vi "UHR-Fleezers Control (host) - 12.7.vi"() -> ()   [LabVIEW 2012] (continued)
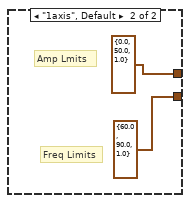
[diagram p2: hidden frame]
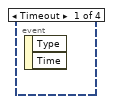
[diagram p3: hidden frame]
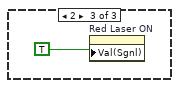
[diagram p6: hidden frame]
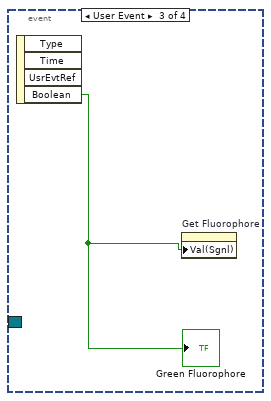
[diagram p7: hidden frame]
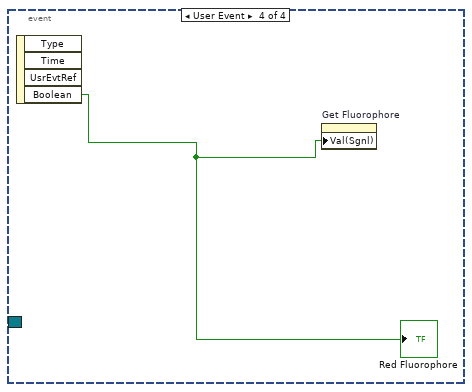
[diagram p8: hidden frame]
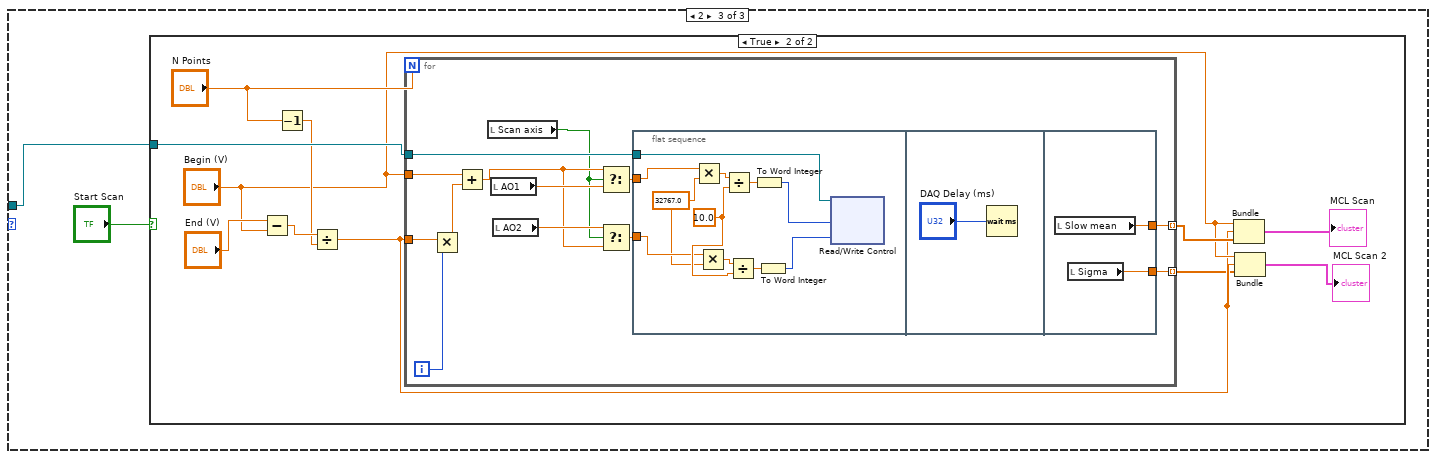
[diagram p10: hidden frame]
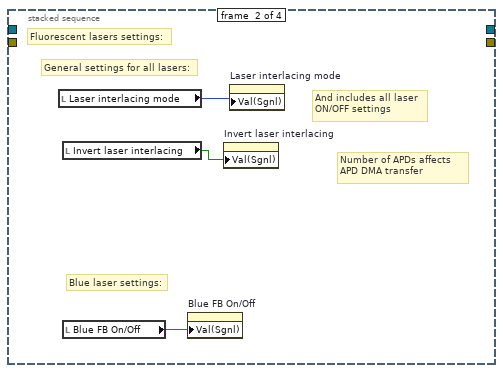
[diagram p12: hidden frame]
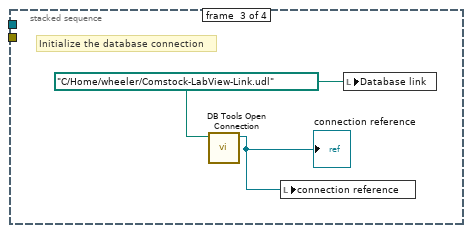
[diagram p13: hidden frame]
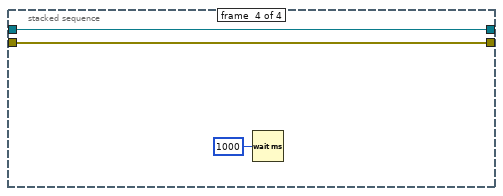
[diagram p14: hidden frame]
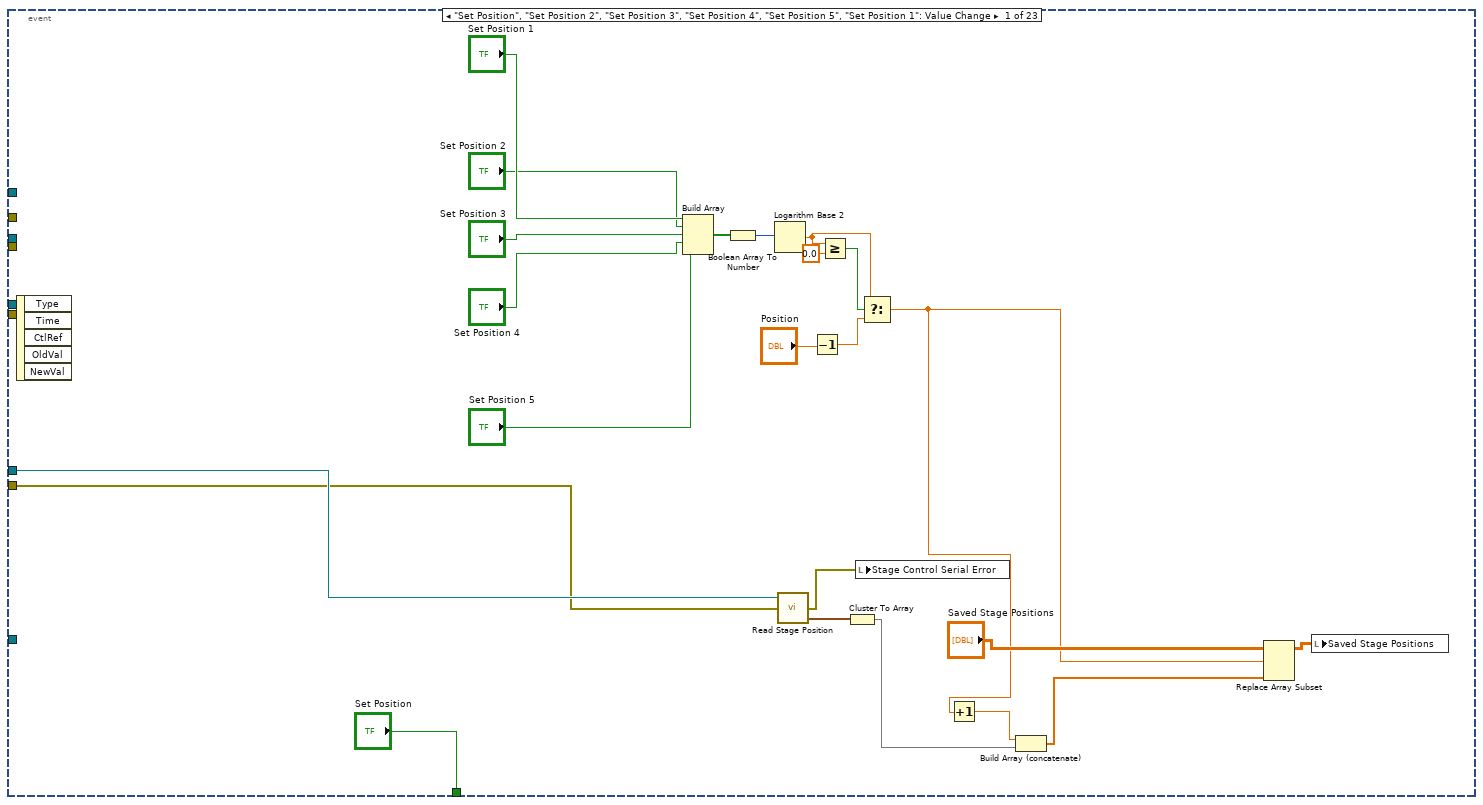
[diagram p16: hidden frame]
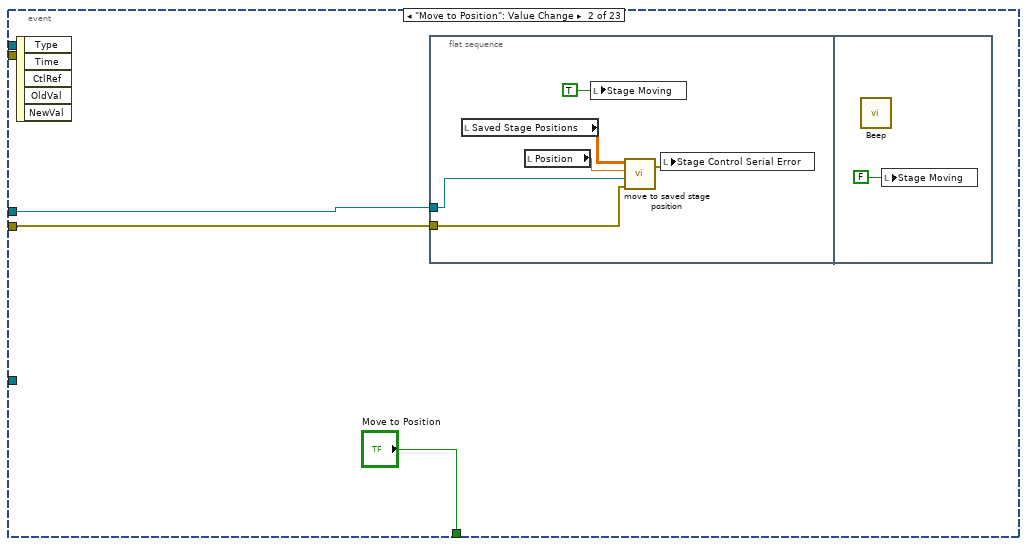
[diagram p17: hidden frame]
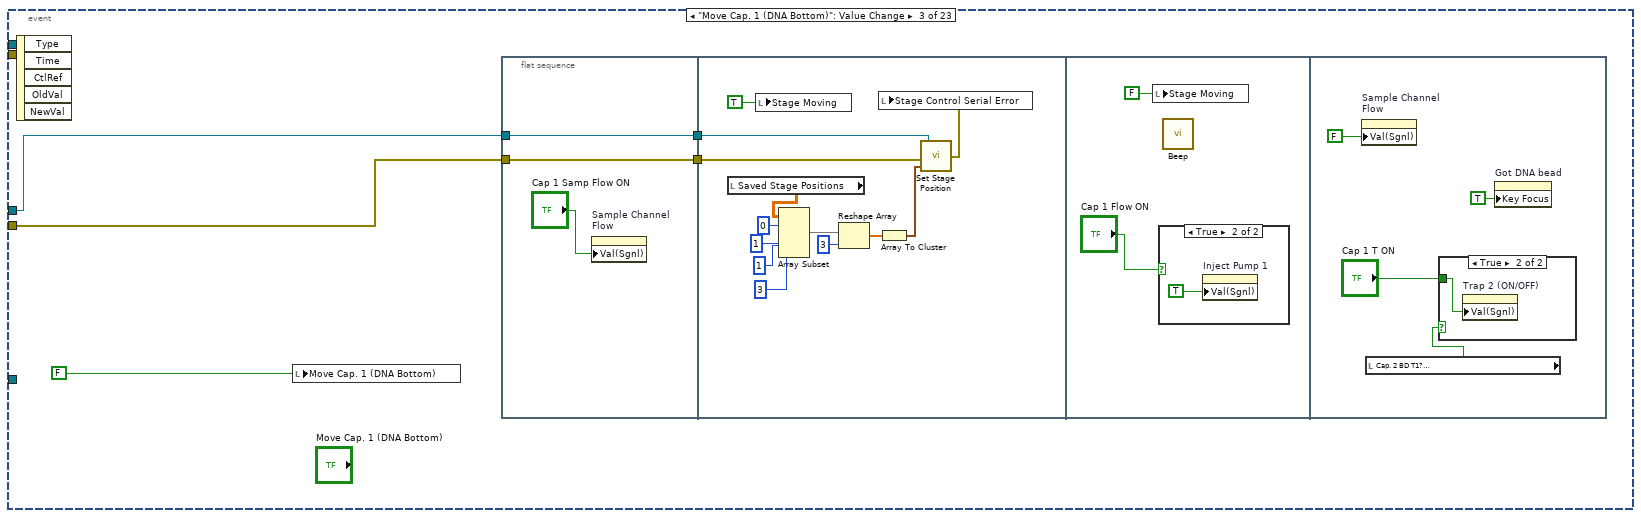
[diagram p18: hidden frame]
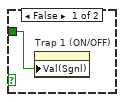
[diagram p20: hidden frame]
              tunnel: [refnum<k0> refnum w4586] -> w4529
              frame False {
              }
              frame True {
                w4585 = 0.0
                n2952 = local read "APD Integration Time (s)"() -> (w4591:dbl)
                n2953 = local read "N APD Samp/step"() -> (w4584:dbl)
                n2954 = local read "Number of APDs"() -> (w4583:u8)
                n2955 = Path To String(path=w4606) -> (string=w4605:string)
                n2956 = String Length(string=w4605) -> (length=w4604:i32)
                n2957 = Subtract(x=w4604, y=4) -> (x-y=w4602:i32)
                n2958 = String Subset(string=w4605, length (rest)=w4602) -> (substring=w4601:string)  [unwired: 1 out]
                n2959 = Build Array(w4591, w4584, w4583, w4585, w4585, w4585, w4585, w4585) -> (w4588:dbl[])
                n2960 = Concatenate Strings(w4601, "_fl.dat" ("string")) -> (w4599:string)
                n2961 = Array Size(array=w4588) -> (size(s)=w4590:i32)
                n2962 = String To Path(string=w4599) -> (path=w4595:path)
                n2963 = Open/Create/Replace File(file path (use dialog)=w4595, operation (0:open)=T29."create", access (0:read/write)=enum16{"read/write", "read-only", "write-only"}."write-only") -> (refnum out=w4596:refnum<file>)  [unwired: 1 in, 4 out]
                n2964 = Deny Access(7:w4596) -> (3:w4592:refnum<file>)  [unwired: 1 in, 2 out]
                n2965 = To Double Precision Float(number=w4590) -> (double precision float=w4589:dbl)
                n2966 = Build Array (concatenate)(w4589, w4588) -> (w4587:dbl[])
                n2967 = Write to Binary File(file (use dialog)=w4592, data=w4587, 5:FALSE ("prepend array or string size? (T)"), 9:T28."big-endian, network order" ("byte order (0:big-endian, network order)")) -> (refnum out=w4586:refnum<file>)  [unwired: 1 in, 3 out]
              }
            }
            n2968 = case shown="True" w4516 {
              tunnel: w4512 -> [_ w4567]
              tunnel: [refnum<k0> refnum w4566] -> w4517
              frame False {
              }
              frame True {
                w4562 = 0.0 ("element")
                n2969 = Path To String(path=w4567) -> (string=w4581:string)
                n2970 = Build Array(w4562, w4562, w4562, w4562, w4562, w4562, w4562, w4562) -> (w4563:dbl[])
                n2971 = String Length(string=w4581) -> (length=w4580:i32)
                n2972 = Subtract(x=w4580, y=4) -> (x-y=w4578:i32)
                n2973 = Array Size(array=w4563) -> (size(s)=w4565:i32)
                n2974 = String Subset(string=w4581, length (rest)=w4578) -> (substring=w4577:string)  [unwired: 1 out]
                n2975 = To Double Precision Float(number=w4565) -> (double precision float=w4564:dbl)
                n2976 = Concatenate Strings(w4577, "_pos.dat" ("string")) -> (w4575:string)
                n2977 = Build Array (concatenate)(w4564, w4563) -> (w4561:dbl[])
                n2978 = String To Path(string=w4575) -> (path=w4571:path)
                n2979 = Open/Create/Replace File(file path (use dialog)=w4571, operation (0:open)=T29."create", access (0:read/write)=enum16{"read/write", "read-only", "write-only"}."write-only") -> (refnum out=w4572:refnum<file>)  [unwired: 1 in, 4 out]
                n2980 = Deny Access(7:w4572) -> (3:w4568:refnum<file>)  [unwired: 1 in, 2 out]
                n2981 = Write to Binary File(file (use dialog)=w4568, data=w4561, 5:FALSE ("prepend array or string size? (T)"), 9:T28."big-endian, network order" ("byte order (0:big-endian, network order)")) -> (refnum out=w4566:refnum<file>)  [unwired: 1 in, 3 out]
              }
            }
            n2982 = Write to Binary File(file (use dialog)=w4552, data=w4511, 5:w4534, 9:w4533) -> (refnum out=w4535:refnum<file>)  [unwired: 1 in, 3 out]
            n2983 = Write to Binary File(file (use dialog)=w4535, data="Comment (data description)", 5:w4534, 9:w4533) -> (refnum out=w4532:refnum<file>)  [unwired: 1 in, 3 out]
            n2984 = local read "connection reference"() -> (w4514:T17)
            n2985 = Bundle("Comment (data description)"="Comment (data description)", "Channel 1 Buffer"="Channel 1 Buffer", "Channel 2 Buffer"="Channel 2 Buffer", "Channel 3 Buffer"="Channel 3 Buffer", "Title"="Title", "DNA Construct"="DNA Construct", "Bead diameter"="Bead diameter", "Name"="Name") -> (w4502:T47)  [unwired: 1 in]
            n2986 = call "MattFileCreator-v9.vi"("Comments"=w4502, "Input Array"=w4511, "File path"=w4512, "table"="labview", "connection reference"=w4514) -> ("connection reference out"=w4513:T17)  [unwired: 5 in, 1 out]
            n2987 = local write "connection reference"(w4513) -> ()
          }
        }
        n2988 = feedback-in #27(w4462) -> ()
        n2989 = feedback-in #28(w4489) -> ()
        n2990 = feedback-in #29(w4461) -> ()
        n2991 = feedback-in #30(w4472) -> ()
        n2992 = feedback-in #31(w4475) -> ()
        n2993 = feedback-in #32(w4488) -> ()
        n2994 = feedback-in #33(w4478) -> ()
      }
      frame #1 {
        n2995 = local read "Saving..."() -> (w4732:bool)
        n2996 = case shown="True" w4732 {
          tunnel: w4736 -> [_ w4747]
          tunnel: w4735 -> [_ w4761]
          tunnel: w4734 -> [_ w4757]
          tunnel: w4733 -> [_ w4756]
          tunnel: w4731 -> [_ w4755]
          tunnel: w4730 -> [_ w4750]
          tunnel: w4729 -> [_ w4749]
          tunnel: w4728 -> [_ w4748]
          tunnel: w4727 -> [_ w4746]
          tunnel: w4726 -> [_ w4744]
          tunnel: w4725 -> [_ w4743]
          tunnel: w4724 -> [_ w4742]
          tunnel: w4723 -> [_ w4741]
          tunnel: w4722 -> [_ w4740]
          tunnel: w4721 -> [_ w4739]
          tunnel: w4720 -> [_ w4738]
          tunnel: w4719 -> [_ w4737]
          frame False {
          }
          frame True {
            n2997 = Multiply(x=w4747, y=w4746) -> (x*y=→"Time (s)":dbl)
            n2998 = Less Or Equal?(x=w4747, y=w4755) -> (x <= y?=w4759:bool)
            n2999 = Or(x="Stop Saving", y="Abort save 2") -> (x .or. y?=w4751:bool)
            n3000 = Not(x=w4751) -> (.not. x?=w4760:bool)
            n3001 = And(x=w4759, y=w4760) -> (x .and. y?=w4758:bool)
            n3002 = case shown="True" w4758 {
              tunnel: w4761 -> [w4768 w4859]
              tunnel: [0.0 w4862] -> w4754
              tunnel: w4747 -> [_ w4860]
              tunnel: w4755 -> [_ w4861]
              tunnel: w4757 -> [_ w4856]
              tunnel: w4756 -> [_ _]
              tunnel: w4750 -> [w4766 w4849]
              tunnel: w4749 -> [w4765 w4850]
              tunnel: w4748 -> [_ w4848]
              tunnel: w4744 -> [_ w4847]
              tunnel: w4743 -> [_ w4771]
              tunnel: w4742 -> [_ w4840]
              tunnel: w4741 -> [_ w4787]
              tunnel: w4740 -> [w4762 w4804]
              tunnel: w4739 -> [w4763 w4803]
              tunnel: w4738 -> [_ w4800]
              tunnel: w4737 -> [_ w4798]
              frame False {
                w4764 = FALSE
                n3003 = Close File(refnum=w4768) -> ()  [unwired: 1 in, 2 out]
                n3004 = case shown="True" w4765 {
                  tunnel: w4766 -> [_ w4770]
                  frame False {
                  }
                  frame True {
                    n3005 = Close File(refnum=w4770) -> ()  [unwired: 1 in, 2 out]
                  }
                }
                n3006 = case shown="True" w4762 {
                  tunnel: w4763 -> [_ w4769]
                  frame False {
                  }
                  frame True {
                    n3007 = Close File(refnum=w4769) -> ()  [unwired: 1 in, 2 out]
                  }
                }
                n3008 = local write "Raster Scanning..."(w4764) -> ()
                n3009 = local write "Calibrating Trap..."(w4764) -> ()
                n3010 = call <vilib>:"Beep.vi"() -> ()  [unwired: 3 in, 9 out]
                n3011 = local write "Stop Saving"(w4764) -> ()
                "Saving..." <- w4764
              }
              frame True {
                n3012 = local read "Calibrating Trap..."() -> (w4851:bool)
                n3013 = case "Write fl. data" shown="True" w4850 {
                  tunnel: w4849 -> [_ w4885]
                  tunnel: w4848 -> [_ w4884]
                  frame False {
                  }
                  frame True {
                    n3014 = Write to Binary File(file (use dialog)=w4885, data=w4884, 5:FALSE ("prepend array or string size? (T)"), 9:T28."big-endian, network order" ("byte order (0:big-endian, network order)")) -> ()  [unwired: 1 in, 4 out]
                  }
                }
                n3015 = Greater?(x="Save ave N", y=1.0) -> (0:w4854:bool)
                n3016 = Not(x=w4851) -> (.not. x?=w4853:bool)
                n3017 = And(x=w4853, y=w4854) -> (x .and. y?=w4801:bool)
                n3018 = case shown="True" w4801 {
                  tunnel: w4800 -> [w4865 w4876]
                  tunnel: [w4865 w4868] -> w4799
                  tunnel: "Save ave N" -> [_ w4869]
                  frame False {
                  }
                  frame True {
                    w4866 = 2 ("dimension size")
                    n3019 = Array Size(array=w4876) -> (size(s)=w4870:i32)
                    n3020 = Divide(x=w4870, y=w4866) -> (x/y=w4874:dbl)
                    n3021 = Reshape Array(w4876, w4874, w4866) -> (w4875:u64[][])
                    n3022 = Transpose 2D Array(2D array=w4875) -> (transposed array=w4873:u64[][])
                    n3023 = for {
                      tunnel: w4873 -> [w4878] mode=indexing
                      tunnel: [w4877] -> w4867 mode=indexing
                      tunnel: w4869 -> [w4879]
                      workers-P: _ -> [_]
                      n3024 = call "downsample 1D array - U64.vi"("Ave N"=w4879, "Array In"=w4878) -> ("Array Out"=w4877:u64[])  [unwired: 1 in]
                    }
                    n3025 = Transpose 2D Array(2D array=w4867) -> (transposed array=w4872:u64[][])
                    n3026 = Divide(x=w4870, y=w4869) -> (x/y=w4871:dbl)
                    n3027 = Reshape Array(w4872, w4871) -> (w4868:u64[])
                  }
                }
                n3028 = case shown="True" w4801 {
                  tunnel: w4856 -> [w4888 w4900]
                  tunnel: [w4888 w4892] -> w4852
                  tunnel: "Save ave N" -> [_ w4893]
                  tunnel: w4847 -> [_ w4891]
                  frame False {
                  }
                  frame True {
                    n3029 = Array Size(array=w4900) -> (size(s)=w4894:i32)
                    n3030 = Array Size(array=w4891) -> (size(s)=w4890:i32)
                    n3031 = Divide(x=w4894, y=w4890) -> (x/y=w4898:dbl)
                    n3032 = Reshape Array(w4900, w4898, w4890) -> (w4899:i16[][])
                    n3033 = Transpose 2D Array(2D array=w4899) -> (transposed array=w4897:i16[][])
                    n3034 = for {
                      tunnel: w4897 -> [w4903] mode=indexing
                      tunnel: [w4902] -> w4889 mode=indexing
                      tunnel: w4893 -> [w4901]
                      workers-P: _ -> [_]
                      n3035 = call "downsample 1D array - I16.vi"("Ave N"=w4901, "Array In"=w4903) -> ("Array Out"=w4902:i16[])  [unwired: 1 out]
                    }
                    n3036 = Transpose 2D Array(2D array=w4889) -> (transposed array=w4896:i16[][])
                    n3037 = Divide(x=w4894, y=w4893) -> (x/y=w4895:dbl)
                    n3038 = Reshape Array(w4896, w4895) -> (w4892:i16[])
                  }
                }
                n3039 = Index Array(array=w4787, index=2) -> (element=w4788:waveform(dbl))
                n3040 = Index Array(array=w4787, index=1) -> (element=w4821:waveform(dbl))
                n3041 = Index Array(array=w4787, index=0) -> (element=w4823:waveform(dbl))
                n3042 = Unbundle By Name(w4788) -> ("Y"=w4790:dbl[])
                n3043 = Unbundle By Name(w4821) -> ("Y"=w4825:dbl[])
                n3044 = Unbundle By Name(w4823) -> ("Y"=w4833:dbl[])
                n3045 = case "Write trap pos. data" shown="True" w4804 {
                  tunnel: w4803 -> [_ w4881]
                  tunnel: w4799 -> [_ w4880]
                  frame False {
                  }
                  frame True {
                    n3046 = Write to Binary File(file (use dialog)=w4881, data=w4880, 5:FALSE ("prepend array or string size? (T)"), 9:T28."big-endian, network order" ("byte order (0:big-endian, network order)")) -> ()  [unwired: 1 in, 4 out]
                  }
                }
                n3047 = Write to Binary File(file (use dialog)=w4859, data=w4852, 5:FALSE ("prepend array or string size? (T)"), 9:T28."big-endian, network order" ("byte order (0:big-endian, network order)")) -> ()  [unwired: 1 in, 4 out]
                n3048 = feedback #34(w4790) -> (w4791:dbl[])
                n3049 = Build Array (concatenate)(w4791, w4790) -> (w4786:dbl[])
                n3050 = Select(t=w4790, s=w4771, f=w4786) -> (s? t:f=w4776:dbl[])
                n3051 = feedback-in #34(w4776) -> ()
                n3052 = feedback #35(w4825) -> (w4827:dbl[])
                n3053 = Build Array (concatenate)(w4827, w4825) -> (w4826:dbl[])
                n3054 = Select(t=w4825, s=w4771, f=w4826) -> (s? t:f=w4815:dbl[])
                n3055 = feedback-in #35(w4815) -> ()
                n3056 = feedback #36(w4833) -> (w4846:dbl[])
                n3057 = Build Array (concatenate)(w4846, w4833) -> (w4845:dbl[])
                n3058 = Select(t=w4833, s=w4771, f=w4845) -> (s? t:f=w4820:dbl[])
                n3059 = feedback-in #36(w4820) -> ()
                n3060 = Divide(x=w4860, y=w4861) -> (x/y=w4863:dbl)
                n3061 = Multiply(x=w4863, y=100.0) -> (x*y=w4862:dbl)
                n3062 = Build Array(w4820, w4815, w4776) -> (→"Saved APD":dbl[][])
                n3063 = Array Size(array=w4820) -> (size(s)=w4838:i32)
                n3064 = Unbundle By Name(w4840) -> ("Y"=w4844:dbl[])
                n3065 = Subtract(x=w4838, y="N pts to average") -> (x-y=w4773:i32)
                n3066 = Multiply(x="N pts to average", y=u16 2) -> (x*y=w4816:u16)
                n3067 = Subtract(x=w4838, y=w4816) -> (x-y=w4774:i32)
                n3068 = feedback #37(w4844) -> (w4843:dbl[])
                n3069 = Build Array (concatenate)(w4843, w4844) -> (w4842:dbl[])
                n3070 = Select(t=w4844, s=w4771, f=w4842) -> (s? t:f=w4841:dbl[])
                "Trap Delta Graph" <- w4841
                n3071 = feedback-in #37(w4841) -> ()
                n3072 = Array Subset(array=w4820, index=w4773, length="N pts to average") -> (w4837:dbl[])
                n3073 = Array Subset(array=w4820, index=w4774, length="N pts to average") -> (w4836:dbl[])
                n3074 = Array Subset(array=w4815, index=w4773, length="N pts to average") -> (w4818:dbl[])
                n3075 = Array Subset(array=w4815, index=w4774, length="N pts to average") -> (w4817:dbl[])
                n3076 = Array Subset(array=w4776, index=w4773, length="N pts to average") -> (w4785:dbl[])
                n3077 = Array Subset(array=w4776, index=w4774, length="N pts to average") -> (w4784:dbl[])
                n3078 = Index Array(array=w4798, index=0) -> (element=w4796:waveform(dbl))
                n3079 = call-poly <vilib>:"Mean.vi"("X"=w4837) -> ("mean"=w4835:dbl)  [unwired: 1 out]
                n3080 = call-poly <vilib>:"Mean.vi"("X"=w4818) -> ("mean"=w4814:dbl)  [unwired: 1 out]
                n3081 = call-poly <vilib>:"Mean.vi"("X"=w4836) -> ("mean"=w4834:dbl)  [unwired: 1 out]
                n3082 = call-poly <vilib>:"Mean.vi"("X"=w4817) -> ("mean"=w4813:dbl)  [unwired: 1 out]
                n3083 = call-poly <vilib>:"Mean.vi"("X"=w4785) -> ("mean"=w4783:dbl)  [unwired: 1 out]
                n3084 = call-poly <vilib>:"Mean.vi"("X"=w4784) -> ("mean"=w4782:dbl)  [unwired: 1 out]
                n3085 = Unbundle By Name(w4796) -> ("Y"=w4794:dbl[])
                n3086 = Subtract(x=w4814, y=w4813) -> (x-y=w4805:dbl)
                "Delta Fl. 2" <- w4805
                n3087 = Subtract(x=w4783, y=w4782) -> (x-y=w4777:dbl)
                "Delta Fl. 3" <- w4777
                n3088 = Subtract(x=w4835, y=w4834) -> (x-y=w4832:dbl)
                "Delta Fl. 1" <- w4832
                n3089 = feedback #38(w4794) -> (w4793:dbl[])
                n3090 = Build Array (concatenate)(w4793, w4794) -> (w4795:dbl[])
                n3091 = Initialize Array(w4832, 1 ("dimension size")) -> (w4829:dbl[])
                n3092 = Initialize Array(w4805, 1 ("dimension size")) -> (w4810:dbl[])
                n3093 = Initialize Array(w4777, 1 ("dimension size")) -> (w4779:dbl[])
                n3094 = Select(t=w4794, s=w4771, f=w4795) -> (s? t:f=w4792:dbl[])
                "Saved trap pos" <- w4792
                n3095 = feedback-in #38(w4792) -> ()
                n3096 = feedback #39(w4829) -> (w4830:dbl[])
                n3097 = Build Array (concatenate)(w4830, w4829) -> (w4828:dbl[])
                n3098 = feedback #40(w4810) -> (w4811:dbl[])
                n3099 = feedback #41(w4779) -> (w4780:dbl[])
                n3100 = Build Array (concatenate)(w4811, w4810) -> (w4809:dbl[])
                n3101 = Build Array (concatenate)(w4780, w4779) -> (w4778:dbl[])
                n3102 = Select(t=w4829, s=w4771, f=w4828) -> (s? t:f=w4808:dbl[])
                n3103 = feedback-in #39(w4808) -> ()
                n3104 = Select(t=w4810, s=w4771, f=w4809) -> (s? t:f=w4807:dbl[])
                n3105 = feedback-in #40(w4807) -> ()
                n3106 = Select(t=w4779, s=w4771, f=w4778) -> (s? t:f=w4772:dbl[])
                n3107 = feedback-in #41(w4772) -> ()
                n3108 = Build Array(w4808, w4807, w4772) -> (→"Save APD Deriv":dbl[][])
              }
            }
            "Progress" <- w4754
            "Progress 2" <- w4754
          }
        }
      }
    }
    n3109 = local read "wait to reset values"() -> (w3406:bool)
    n3110 = Not(x=w3404) -> (.not. x?=w3407:bool)
    n3111 = And(x=w3407, y=w3406) -> (x .and. y?=w3408:bool)
    n3112 = case "Part of MCL raster scanning: returns to initial positions after scan done" shown="True" w3408 {
      tunnel: w3139 -> [w4282 w4289]
      tunnel: [w4282 w4288] -> w3410
      tunnel: w3138 -> [w4281 w4287]
      tunnel: [w4281 w4286] -> w3405
      frame False {
      }
      frame True {
        w4297 = 10.0 ("y")
        w4296 = 32767.0 ("y")
        # "to return scan values\nafter a synchronous \nAOM scan"
        n3113 = local read "AO2"() -> (w4290:dbl)
        n3114 = local read "AO1"() -> (w4291:dbl)
        n3115 = local write "wait to reset values"(FALSE ("wait to reset values")) -> ()
        n3116 = Multiply(x=w4291, y=w4296) -> (x*y=w4293:dbl)
        n3117 = Multiply(x=w4290, y=w4296) -> (x*y=w4295:dbl)
        n3118 = Divide(x=w4293, y=w4297) -> (x/y=w4292:dbl)
        n3119 = Divide(x=w4295, y=w4297) -> (x/y=w4294:dbl)
        n3120 = To Word Integer(number=w4292) -> (16bit integer=w4298:i16)
        n3121 = To Word Integer(number=w4294) -> (16bit integer=w4299:i16)
        n3122 = local read "Total Counts (ticks)"() -> (w4283:u16)
        n3123 = xnode "Read/Write Control"("FPGA VI Reference In"=w4289, "error in"=w4287, "AO1"=w4298, "AO2"=w4299, "MCL count"=w4283) -> ("FPGA VI Reference Out"=w4288:T20, "error out"=w4286:errorcluster)
        n3124 = local read "Scan Range (V)\n(of steps)"() -> (w4284:dbl)
        n3125 = property on="Scan Range (V)\n(of steps)" class="DigNum (strict)"("Val(Sgnl)"=w4284) -> ()  [unwired: 2 in, 2 out]
      }
    }
    n3126 = node-c288() -> ()  [unwired: 2 out]
  }
  n3127 = flat-sequence "Video" {
    tunnel: [w4913] -> w116
    tunnel: w116 -> [w4953]
    frame #0 {
      n3128 = while {
        stop <- w4905 continue-if-true
        n3129 = call "Close Video Capture.vi"() -> ("error code OUT"=w4907:i32)
        n3130 = Equal?(x=w4907, y=0) -> (x = y?=w4905:bool)
      }
      n3131 = local write "Stop All"(FALSE ("Stop All")) -> ()
    }
    frame #1 {
      n3132 = call "DMR_Init.vi"() -> ()  [unwired: 3 out]
    }
    frame #2 {
      w4908 = "DE245428202"  # MSU fleezers card #
      (unwired) "DE019116701"  # Illinois fleezers card #
      # "Setting the destination format to Mono8 makes sure that the image can be displayed in the intensity plot."
      n3133 = call "DMR_GetDevice.vi"("search string IN"=w4908) -> ("device handle OUT"=w4931:i32)  [unwired: 4 in, 2 out]
      n3134 = call "DMR_OpenDevice.vi"("device handle IN"=w4931) -> ("driver handle OUT"=w4914:i32)  [unwired: 4 out]
      n3135 = call "DMR_FindList.vi"("flags IN"=u32 0 ("flags"), "list name IN"="" ("String"), "list type IN"=T48."camera descriptions", "driver handle IN"=w4914) -> ("list handle OUT"=w4917:i32)  [unwired: 2 out]
      n3136 = call "DMR_FindList.vi"("flags IN"=u32 0 ("flags"), "list name IN"="Base", "list type IN"=T48."setting", "driver handle IN"=w4914) -> ("list handle OUT"=w4915:i32)  [unwired: 2 out]
      n3137 = call "OBJ_GetHandle.vi"("object name IN"="VideoStandard", "list handle IN"=w4917) -> ("object handle OUT"=w4911:i32)  [unwired: 3 out]
      n3138 = call "OBJ_GetHandle.vi"("object name IN"="PixelFormat", "list handle IN"=w4915) -> ("object handle OUT"=w4925:i32)  [unwired: 3 out]
      n3139 = call "OBJ_SetS.vi"("value index IN"=0, "value IN"="NTSC M", "object handle IN"=w4911) -> ()  [unwired: 2 out]
      n3140 = call "OBJ_SetS.vi"("value index IN"=0, "value IN"="Mono8" ("value"), "object handle IN"=w4925) -> ()  [unwired: 2 out]
      n3141 = call "OBJ_GetHandle.vi"("object name IN"="VideoChannel", "list handle IN"=w4915) -> ("object handle OUT"=w4921:i32)  [unwired: 3 out]
      n3142 = while {
        tunnel: [w4935] -> w4913
        tunnel: w4914 -> [w4932]
        stop <- w4933 continue-if-true
        n3143 = call "DMR_ImageRequestSingle.vi"("request control IN"=0, "driver handle IN"=w4932) -> ("error code OUT"=w4934:i32, "driver handle OUT"=w4935:i32)  [unwired: 2 out]
        n3144 = Equal To 0?(x=w4934) -> (x = 0?=w4933:bool)
      }
      n3145 = call "OBJ_SetI.vi"("value index IN"=0, "value IN"=3 ("Video channel"), "object handle IN"=w4921) -> ()  [unwired: 2 out]
    }
    frame #3 {
      w4941 = T18 0 items=["Grayscale (U8)", "Grayscale (I16)", "Grayscale (SGL)", "Complex (CSG)", "RGB (U32)", "HSL (U32)", "RGB (U64)"] ("Image Type")
      w4949 = T18 0 items=["Grayscale (U8)", "Grayscale (I16)", "Grayscale (SGL)", "Complex (CSG)", "RGB (U32)", "HSL (U32)", "RGB (U64)"] ("Image Type")
      n3146 = for "Create Greyscale map" {
        N: 256 -> [_]
        tunnel: [w4955] -> w4938 mode=indexing
        workers-P: _ -> [_]
        i -> [w4958]
        n3147 = To Unsigned Byte Integer(number=w4958) -> (unsigned 8bit integer=w4954:u8)
        n3148 = Join Numbers(hi=w4954, lo=w4954) -> ((hi.lo)=w4957:u16)
        n3149 = Join Numbers(hi=w4954, lo=w4954) -> ((hi.lo)=w4956:u16)
        n3150 = Join Numbers(hi=w4957, lo=w4956) -> ((hi.lo)=w4955:u32)
      }
      n3151 = call "IMAQ Create"("Image Name"="Scaled video", "Image Type"=w4941) -> ("New Image"=w4940:T2)  [unwired: 2 in, 2 out]
      n3152 = call "IMAQ Create"("Image Name"="Main video", "Image Type"=w4949) -> ("New Image"=w4950:T2)  [unwired: 2 in, 2 out]
      n3153 = node-c288(0 ("Processor")) -> (w4948:T23)  [unwired: 3 out]
      n3154 = Initialize Array(u32 0 ("Window Number (0...15)"), 480 ("dimension size"), 640 ("dimension size")) -> (w4943:u32[][])
      n3155 = timed-loop {
        tunnel: w4953 -> [w4975]
        tunnel: [w4974] -> w4952
        tunnel: w4950 -> [w4973]
        timing: w4948 -> [_]
        timing-out: [_] -> w4947
        tunnel: w4943 -> [w4962]
        tunnel: w4940 -> [w4960]
        tunnel: w4938 -> [w4959]
        stop <- w4961 stop-if-true
        # "This block performs the \nactual image capture."
        n3156 = node-c288() -> ()  [unwired: 2 out]
        n3157 = local read "Stop All"() -> (w4961:bool)
        n3158 = Reciprocal(x="Video Capture Rate (Hz)") -> (1/x=w4965:dbl)
        n3159 = Multiply(x=w4965, y=1000.0) -> (x*y=w4963:dbl)
        n3160 = call "DMR_ImageRequestWaitFor.vi"("queue number IN"=0, "timeout(ms) IN"=500, "driver handle IN"=w4975) -> ("error code OUT"=w4979:i32, "request number OUT"=w4976:i32, "driver handle OUT"=w4977:i32)
        n3161 = feedback #42(T49 refnum ("Avi Refnum")) -> (w4967:T49)
        n3162 = case shown="True" "New Video File" {
          tunnel: [T49 refnum ("Avi Refnum") w4996] -> w4969
          tunnel: [FALSE TRUE] -> w4970
          tunnel: w4967 -> [_ w4992]
          frame False {
          }
          frame True {
            n3163 = call "Create new save file.vi"("Ext"=".avi" ("string"), "Index In"="Video Index") -> ("Path Out"=w4988:path, "Index Out"=w4989:dbl)  [unwired: 1 in]
            "Path Out" <- w4988
            n3164 = Not Equal?(x=w4992, y=T49 refnum ("Avi Refnum")) -> (x != y?=w4993:bool)
            n3165 = Increment(x=w4989) -> (x+1=w4998:dbl)
            n3166 = case shown="True" w4993 {
              tunnel: w4992 -> [_ w4999]
              frame False {
              }
              frame True {
                n3167 = call "IMAQ AVI Close"("Avi Refnum"=w4999) -> ()  [unwired: 1 in, 10 out]
              }
            }
            n3168 = local write "Video Index"(w4998) -> ()
            n3169 = call "IMAQ AVI Create"("Frames Per Second"=u32 30, "AVI Path"=w4988) -> ("Avi Refnum"=w4996:T49)  [unwired: 5 in, 4 out]
          }
        }
        n3170 = Equal To 0?(x=w4979) -> (x = 0?=w4978:bool)
        n3171 = Select(t=w4969, s=w4970, f=w4967) -> (s? t:f=w4968:T49)
        n3172 = feedback-in #42(w4968) -> ()
        n3173 = case shown="True" w4978 {
          tunnel: w4977 -> [w5000 w5034]
          tunnel: w4976 -> [_ w5033]
          tunnel: [w5000 w5030] -> w4974
          tunnel: w4973 -> [_ w5015]
          tunnel: w4962 -> [_ w5019]
          tunnel: w4968 -> [_ w5017]
          tunnel: w4960 -> [_ w5012]
          tunnel: w4959 -> [_ w5011]
          frame False {
          }
          frame True {
            w5024 = u32 0 ("X-offset IN")
            n3174 = call "DMR_GetImageRequestBufferData.vi"("driver handle IN"=w5034, "request number IN"=w5033) -> ("width OUT"=w5023:i32, "height OUT"=w5022:i32, "driver handle OUT"=w5029:i32, "request number OUT"=w5028:i32, "bytes per pixel OUT"=w5025:i32)  [unwired: 13 out]
            n3175 = call "DMR_GetImageRequestBufferImageData.vi"("driver handle IN"=w5029, "request number IN"=w5028, "bytes per pixel IN"=w5025, "X-offset IN"=w5024, "Y-offset IN"=w5024, "height IN"=w5022, "width IN"=w5023) -> ("driver handle OUT"=w5027:u32, "request number OUT"=w5026:u32, "image OUT"=w5004:u32[][])  [unwired: 10 out]
            n3176 = Transpose 2D Array(2D array=w5004) -> (transposed array=w5010:u32[][])
            n3177 = Select(t=w5010, s="Flip Y (or X)", f=w5004) -> (s? t:f=w5009:u32[][])
            n3178 = call "DMR_ImageRequestUnlock.vi"("request number IN"=w5026, "driver handle IN"=w5027) -> ("driver handle OUT"=w5032:i32)  [unwired: 1 in, 2 out]
            n3179 = for {
              tunnel: w5009 -> [w5069] mode=indexing
              tunnel: [w5068] -> w5007 mode=indexing
              n3180 = Reverse 1D Array(array=w5069) -> (reversed array=w5068:u32[])
            }
            n3181 = call "DMR_ImageRequestSingle.vi"("request control IN"=0, "driver handle IN"=w5032) -> ("driver handle OUT"=w5030:i32)  [unwired: 3 out]
            n3182 = Transpose 2D Array(2D array=w5007) -> (transposed array=w5008:u32[][])
            n3183 = Select(t=w5008, s="Flip Y (or X)", f=w5007) -> (s? t:f=w5005:u32[][])
            n3184 = Select(t=w5005, s="Flip Image", f=w5004) -> (s? t:f=w5002:u32[][])
            n3185 = case shown="True" "Averaging" {
              tunnel: w5002 -> [w5072 w5077]
              tunnel: [w5072 w5076] -> w5016
              tunnel: w5019 -> [_ w5074]
              frame False {
              }
              frame True {
                (unwired) 1
                w5082 = 1
                n3186 = feedback #43(w5074) -> (w5073:u32[][])
                n3187 = Add(x=w5077, y=w5073) -> (x+y=w5078:u32[][])
                n3188 = Select(t=w5074, s="Reset Averaging", f=w5078) -> (s? t:f=w5080:u32[][])
                n3189 = feedback-in #43(w5080) -> ()
                n3190 = feedback #44(w5082) -> (w5075:i32)
                n3191 = Divide(x=w5078, y=w5075) -> (x/y=w5079:dbl[][])
                n3192 = Increment(x=w5075) -> (x+1=w5083:i32)
                n3193 = To Unsigned Long Integer(number=w5079) -> (unsigned 32bit integer=w5076:u32[][])
                n3194 = Select(t=w5082, s="Reset Averaging", f=w5083) -> (s? t:f=w5081:i32)
                n3195 = feedback-in #44(w5081) -> ()
              }
            }
            n3196 = case shown="True" "Zoom video window" {
              tunnel: w5016 -> [_ w5048]
              tunnel: w5012 -> [_ w5047]
              frame False {
              }
              frame True {
                n3197 = To Double Precision Float(number=w5048) -> (double precision float=w5045:dbl[][])
                n3198 = In Range and Coerce(upper limit="Intensity Upper", x=w5045, lower limit="Intensity Lower") -> (coerced(x)=w5044:dbl[][])  [unwired: 1 out]
                n3199 = Subtract(x="Intensity Upper", y="Intensity Lower") -> (x-y=w5041:dbl)
                n3200 = Subtract(x=w5044, y="Intensity Lower") -> (x-y=w5042:dbl[][])
                n3201 = Divide(x=w5042, y=w5041) -> (x/y=w5043:dbl[][])
                n3202 = Multiply(x=255.0, y=w5043) -> (x*y=w5039:dbl[][])
                n3203 = To Unsigned Byte Integer(number=w5039) -> (unsigned 8bit integer=w5046:u8[][])
                n3204 = call "IMAQ ArrayToImage"("Image Pixels (U8)"=w5046, "Image"=w5047) -> ("Image Out"=w5035:T2)  [unwired: 4 in, 5 out]
                n3205 = First Call?() -> (First Call?: T/F=w5036:bool)
                n3206 = case shown="True" w5036 {
                  tunnel: w5035 -> [w5049 w5060]
                  frame False {
                    n3207 = flat-sequence {
                      tunnel: w5049 -> [w5055]
                      frame #0 {
                        w5052 = FALSE ("Get/Set Status? (Set)")
                        w5051 = 0 ("Window Number (0...15)")
                        n3208 = call "IMAQ WindSize"("Get/Set Status? (Set)"=w5052, "Window Number"=w5051) -> ("Width & Height out"=→"Window Size":cluster{"Width":i32, "Height":i32})  [unwired: 4 in, 2 out]
                        n3209 = call "IMAQ WindMove"("Window Number (0...15)"=w5051, "Get/Set Status? (Set)"=w5052) -> ("Coordinates (screen)"=→"Window Position":cluster{"X Position":i32, "Y Position":i32})  [unwired: 3 in, 1 out]
                        n3210 = call "IMAQ WindDraw"("Resize to Image Size? (Y)"=FALSE, "Window Number (0...15)"=w5051, "Image"=w5055) -> ()  [unwired: 7 in, 2 out]
                      }
                      frame #1 {
                        n3211 = call "IMAQ WindZoom 2"("Center Point"="Center Point", "Zoom to Fit? (False)"=FALSE, "Zoom Factor"="Zoom Factor") -> ()  [unwired: 5 in, 4 out]
                      }
                    }
                  }
                  frame True {
                    n3212 = flat-sequence {
                      tunnel: w5060 -> [w5063]
                      tunnel: [w5061] -> w5059
                      tunnel: w5059 -> [w5065]
                      frame #0 {
                        w5062 = TRUE ("Resize to Image Size? (Y)")
                        w5061 = 0 ("Window Number (0...15)")
                        n3213 = call "IMAQ WindNonTearing"("Window Number"=w5061, "NonTearing? (True)"=w5062) -> ()  [unwired: 8 in, 2 out]
                        n3214 = call "IMAQ WindDraw"("Resize to Image Size? (Y)"=w5062, "Window Number (0...15)"=w5061, "Image"=w5063) -> ()  [unwired: 7 in, 2 out]
                      }
                      frame #1 {
                        n3215 = call "IMAQ WindSize"("Scrollbars? (N)"=FALSE, "Width & Height"="Initial Window Size", "Window Number"=w5065) -> ()  [unwired: 3 in, 3 out]
                        n3216 = call "IMAQ WindMove"("Window Number (0...15)"=w5065, "Coordinates (screen)"="Initial Window Position") -> ()  [unwired: 3 in, 2 out]
                      }
                    }
                  }
                }
              }
            }
            n3217 = To Unsigned Byte Integer(number=w5016) -> (unsigned 8bit integer=w5014:u8[][])
            n3218 = call "IMAQ ArrayToImage"("Image Pixels (U8)"=w5014, "Image"=w5015) -> ("Image Out"=w5013:T2)  [unwired: 4 in, 5 out]
            "Primary Video Display" <- w5013
            n3219 = case shown="True" "Save Video" {
              tunnel: w5017 -> [_ w5071]
              tunnel: w5013 -> [_ w5070]
              frame False {
              }
              frame True {
                n3220 = call "IMAQ AVI Write Frame"("Image"=w5070, "Avi Refnum"=w5071) -> ()  [unwired: 2 in, 8 out]
              }
            }
            n3221 = case shown="True" "Save Image" {
              tunnel: w5014 -> [_ w5086]
              tunnel: w5011 -> [_ w5085]
              frame False {
              }
              frame True {
                n3222 = call <vilib>:"Flatten Pixmap.vi"("colors"=w5085, "8-bit pixmap"=w5086) -> ("image data"=w5092:T50)  [unwired: 4 in, 5 out]
                n3223 = call "Create new save file.vi"("Insert"="video_frame_" ("string"), "Ext"=".bmp" ("string"), "Index In"="Image Index") -> ("Path Out"=w5088:path, "Index Out"=w5093:dbl)
                n3224 = Increment(x=w5093) -> (x+1=w5087:dbl)
                n3225 = local write "Image Index"(w5087) -> ()
                n3226 = call <vilib>:"Write BMP File.vi"("image data"=w5092, "path to BMP file"=w5088) -> ()  [unwired: 1 in, 9 out]
              }
            }
          }
        }
        n3227 = node-c288(w4963) -> ()  [unwired: 1 out]
      }
      n3228 = node-c288(w4947) -> ()  [unwired: 1 out]
      n3229 = call "DMR_CloseDevice.vi"("driver handle IN"=w4952) -> ()  [unwired: 1 in, 4 out]
    }
    frame #4 {
      n3230 = call "DMR_Close.vi"() -> ()  [unwired: 1 out]
    }
  }
  n3231 = timed-loop "Rough control of MCL mirror stage (debugging)" {
    tunnel: w18 -> [w5100]
    tunnel: [w5099] -> w256
    timing: w12 -> [_]
    timing-out: [_] -> w11
    stop <- w5099 stop-if-true
    n3232 = node-c288() -> ()  [unwired: 2 out]
    n3233 = case shown="1" "MCL Mode" {
      tunnel: w5100 -> [_ w5103 w5150]
      frame 0, Default {
      }
      frame 1 {
        n3234 = node-c288() -> (w5105:T23)  [unwired: 4 out]
        n3235 = timed-loop "Oscillate MCL mirror" {
          timing: w5105 -> [_]
          timing-out: [_] -> w5104
          tunnel: w5103 -> [w5144]
          i -> [w5143]
          stop <- w5106 stop-if-true
          n3236 = node-c288() -> (w5142:i64)  [unwired: 1 out]
          n3237 = Multiply(x="AO1", y=32767.0) -> (x*y=w5138:dbl)
          n3238 = Multiply(x="AO2", y=32767.0) -> (x*y=w5133:dbl)
          n3239 = Divide(x=w5138, y=10.0) -> (x/y=w5139:dbl)
          n3240 = Divide(x=w5133, y=10.0) -> (x/y=w5134:dbl)
          n3241 = To Word Integer(number=w5139) -> (16bit integer=w5131:i16)
          n3242 = To Word Integer(number=w5134) -> (16bit integer=w5130:i16)
          n3243 = Divide(x=w5142, y=i64 1000) -> (x/y=w5113:dbl)
          n3244 = Multiply(x=w5113, y=w5143) -> (x*y=w5124:dbl)
          n3245 = Multiply(x="Osc. freq. (Hz) 2", y=6.283185307179586) -> (x*y=w5125:dbl)
          n3246 = Multiply(x=w5125, y=w5124) -> (x*y=w5123:dbl)
          n3247 = Sine(x=w5123) -> (sin(x)=w5122:dbl)
          n3248 = Multiply(x=w5122, y="Osc. amp. (V)") -> (x*y=w5120:dbl)
          n3249 = Add(x=w5120, y="Osc. center (V)") -> (x+y=w5118:dbl)
          n3250 = Divide(x=w5118, y=10.0) -> (x/y=w5116:dbl)
          n3251 = Multiply(x=w5116, y=32767.0) -> (x*y=w5111:dbl)
          n3252 = Select(t=w5111, s="Scan axis", f=w5131) -> (s? t:f=w5129:dbl)
          n3253 = Select(t=w5130, s="Scan axis", f=w5111) -> (s? t:f=w5128:dbl)
          n3254 = local read "MCL Mode"() -> (w5110:u16)
          n3255 = Not Equal?(x=w5110, y=u16 1) -> (x != y?=w5107:bool)
          n3256 = local read "Stop All"() -> (w5108:bool)
          n3257 = xnode "Read/Write Control"("FPGA VI Reference In"=w5144, "AO1"=w5129, "AO2"=w5128) -> ()  [unwired: 1 in, 2 out]
          n3258 = Compound Arithmetic op=OR(w5108, w5107) -> (w5106:bool)
          n3259 = node-c288() -> ()  [unwired: 2 out]
        }
        n3260 = node-c288(w5104) -> ()  [unwired: 1 out]
      }
      frame 2 {
        n3261 = case shown="True" "Start Scan" {
          tunnel: w5150 -> [_ w5162]
          frame False {
          }
          frame True {
            n3262 = Subtract(x="End (V)", y="Begin (V)") -> (x-y=w5158:dbl)
            n3263 = Decrement(x="N Points") -> (x-1=w5157:dbl)
            n3264 = Divide(x=w5158, y=w5157) -> (x/y=w5155:dbl)
            n3265 = for {
              N: "N Points" -> [_]
              tunnel: "Begin (V)" -> [w5175]
              tunnel: w5162 -> [w5167]
              tunnel: [w5166] -> w5161 mode=indexing
              tunnel: w5155 -> [w5165]
              tunnel: [w5163] -> w5154 mode=indexing
              i -> [w5174]
              n3266 = Multiply(x=w5165, y=w5174) -> (x*y=w5173:dbl)
              n3267 = Add(x=w5175, y=w5173) -> (x+y=w5170:dbl)
              n3268 = local read "Scan axis"() -> (w5164:bool)
              n3269 = local read "AO1"() -> (w5172:dbl)
              n3270 = local read "AO2"() -> (w5171:dbl)
              n3271 = Select(t=w5170, s=w5164, f=w5172) -> (s? t:f=w5169:dbl)
              n3272 = Select(t=w5171, s=w5164, f=w5170) -> (s? t:f=w5168:dbl)
              n3273 = flat-sequence {
                tunnel: w5169 -> [w5179]
                tunnel: w5168 -> [w5178]
                tunnel: w5167 -> [w5176]
                tunnel: [w5189] -> w5166
                tunnel: [w5188] -> w5163
                frame #0 {
                  w5182 = 10.0 ("y")
                  w5177 = 32767.0 ("y")
                  n3274 = Multiply(x=w5179, y=w5177) -> (x*y=w5185:dbl)
                  n3275 = Multiply(x=w5178, y=w5177) -> (x*y=w5183:dbl)
                  n3276 = Divide(x=w5185, y=w5182) -> (x/y=w5186:dbl)
                  n3277 = Divide(x=w5183, y=w5182) -> (x/y=w5184:dbl)
                  n3278 = To Word Integer(number=w5186) -> (16bit integer=w5180:i16)
                  n3279 = To Word Integer(number=w5184) -> (16bit integer=w5181:i16)
                  n3280 = xnode "Read/Write Control"("FPGA VI Reference In"=w5176, "AO1"=w5180, "AO2"=w5181) -> ()  [unwired: 1 in, 2 out]
                }
                frame #1 {
                  n3281 = Wait (ms)(milliseconds to wait="DAQ Delay (ms)") -> ()  [unwired: 1 out]
                }
                frame #2 {
                  n3282 = local read "Slow mean"() -> (w5189:dbl)
                  n3283 = local read "Sigma"() -> (w5188:dbl)
                }
              }
            }
            n3284 = Bundle("Begin (V)"="Begin (V)", w5155, w5161) -> (→"MCL Scan":cluster{"Begin (V)":dbl, dbl, dbl[]})  [unwired: 1 out]
            n3285 = Bundle("Begin (V)"="Begin (V)", w5155, w5154) -> (→"MCL Scan 2":cluster{"Begin (V)":dbl, dbl, dbl[]})  [unwired: 1 out]
          }
        }
      }
    }
    n3286 = local read "Stop All"() -> (w5099:bool)
    n3287 = node-c288() -> ()  [unwired: 2 out]
  }
  n3288 = node-c288(w11) -> ()  [unwired: 1 out]
  n3289 = node-c288(w127) -> ()  [unwired: 1 out]
  n3290 = node-c288(w129) -> ()  [unwired: 1 out]
  n3291 = property on="Saved trap pos" class="WFGraph (strict)"("Visible"=FALSE) -> ()  [unwired: 2 in, 2 out]
  n3292 = property on="Trap Delta Graph" class="WFGraph (strict)"("Visible"=TRUE) -> ()  [unwired: 2 in, 2 out]
  n3293 = node-c288(w114) -> ()  [unwired: 1 out]
  n3294 = local write "Trap pos"(FALSE ("Trap pos")) -> ()
  n3295 = disable-structure shown="Disabled" {
    disable-tunnel: w118 -> [w5191 _]
    disable-tunnel: w117 -> [w5190 _]
    frame Disabled {
      n3296 = VISA Close(VISA resource name=w5191, error in (no error)=w5190) -> (error out=w5192:errorcluster)
      n3297 = call <vilib>:"Simple Error Handler.vi"("error in (no error)"=w5192) -> ()  [unwired: 1 in, 8 out]
    }
    frame Enabled {
    }
  }
  n3298 = node-c288(w125) -> ()  [unwired: 1 out]
  n3299 = node-c288(w200) -> ()  [unwired: 1 out]
  n3300 = flat-sequence {
    tunnel: w291 -> [w5196]
    tunnel: w293 -> [w5197]
    tunnel: [w5195] -> w272
    tunnel: [w5194] -> w271
    tunnel: w256 -> [_]
    tunnel: w208 -> [_]
    tunnel: w131 -> [_]
    tunnel: w272 -> [w5198]
    tunnel: w271 -> [w5199]
    frame #0 {
      w5193 = FALSE ("AI to FIFO")
      n3301 = xnode "Read/Write Control"("FPGA VI Reference In"=w5197, "error in"=w5196, "AI to FIFO"=w5193, "APD to FIFO"=w5193) -> ("FPGA VI Reference Out"=w5195:T20, "error out"=w5194:errorcluster)
    }
    frame #1 {
      n3302 = xnode "Close FPGA VI Reference"("FPGA VI Reference In"=w5198, "error in"=w5199) -> ("error out"=→"error out":errorcluster)
    }
  }
